vi "USRP-2945-2955 AoA Detection RX Localization using MUSIC.vi"() -> ()   [LabVIEW 2015] (continued)
  out "USRP error out":errorcluster
  out "Queue error out":errorcluster={"status"=TRUE, "code"=1, "source"="Dequeue Element in USRP-2945-2955 AoA Detection RX Localization using MUSIC (manual phase input).vi"}
  out "# elements in queue (it should keep 0)":i32
  out "coerced IQ rate":dbl=1000000.0 format="%#_6p"
  out "coerced carrier frequency":dbl=462651999.98859316 format="%#_6p"
  out "Eigenvalues":cdb[][](array[numeric])=[[1.4802185041005208e-08+5.36819667616762e-26i], [1.1697264580906096e-08+6.7532415852242355e-25i], [1.006365203344385e-08+3.1450001473342563e-25i], [9.127178536995344e-09+1.972647788120172e-25i]]
  out "The number of sources":i32
  out "Ch 1":cdb[](array[numeric])
  out "Ch 2":cdb[](array[numeric])
  out "Ch 3":cdb[](array[numeric])
  out "Ch 4":cdb[](array[numeric])
  in  "Threshold":dbl=0.001
  in  "Filter":string(combo)="IIR"
  in  "Device Name":refnum<k15>="RIO0"
  in  "Gain":dbl=50.0
  in  "Carrier Frequency":dbl=462652000.0 format="%#_6p"
  in  "IQ Rate":dbl=1000000.0 format="%#_6p"
  in  "Samples per Frame":i32=100000
  in  "Samples used":i32=1000
  in  "Stop":bool
  out "Direction":dbl(knob)=54.0 scale=0.0..180.0
  out "MuSIC spectrum":cluster{"Y":dbl[], "Y":dbl[]}[](graph)=[{"Y"=[0.0, 0.5, 1.0, 1.5, 2.0, 2.5, 3.0, 3.5, 4.0, 4.5, 5.0, 5.5, 6.0, 6.5, 7.0, 7.5, 8.0, 8.5, 9.0, 9.5, 10.0, 10.5, 11.0, 11.5, 12.0, 12.5, 13.0, 13.5, 14.0, 14.5, 15.0, 15.5, 16.0, 16.5, 17.0, 17.5, 18.0, 18.5, 19.0, 19.5, 20.0, 20.5, 21.0, 21.5, 22.0, 22.5, 23.0, 23.5, 24.0, 24.5, 25.0, 25.5, 26.0, 26.5, 27.0, 27.5, 28.0, 28.5, 29.0, 29.5, 30.0, 30.5, 31.0, 31.5, 32.0, 32.5, 33.0, 33.5, 34.0, 34.5, 35.0, 35.5, 36.0, 36.5, 37.0, 37.5, 38.0, 38.5, 39.0, 39.5, 40.0, 40.5, 41.0, 41.5, 42.0, 42.5, 43.0, 43.5, 44.0, 44.5, 45.0, 45.5, 46.0, 46.5, 47.0, 47.5, 48.0, 48.5, 49.0, 49.5, 50.0, 50.5, 51.0, 51.5, 52.0, 52.5, 53.0, 53.5, 54.0, 54.5, 55.0, 55.5, 56.0, 56.5, 57.0, 57.5, 58.0, 58.5, 59.0, 59.5, 60.0, 60.5, 61.0, 61.5, 62.0, 62.5, 63.0, 63.5, 64.0, 64.5, 65.0, 65.5, 66.0, 66.5, 67.0, 67.5, 68.0, 68.5, 69.0, 69.5, 70.0, 70.5, 71.0, 71.5, 72.0, 72.5, 73.0, 73.5, 74.0, 74.5, 75.0, 75.5, 76.0, 76.5, 77.0, 77.5, 78.0, 78.5, 79.0, 79.5, 80.0, 80.5, 81.0, 81.5, 82.0, 82.5, 83.0, 83.5, 84.0, 84.5, 85.0, 85.5, 86.0, 86.5, 87.0, 87.5, 88.0, 88.5, 89.0, 89.5, 90.0, 90.5, 91.0, 91.5, 92.0, 92.5, 93.0, 93.5, 94.0, 94.5, 95.0, 95.5, 96.0, 96.5, 97.0, 97.5, 98.0, 98.5, 99.0, 99.5, 100.0, 100.5, 101.0, 101.5, 102.0, 102.5, 103.0, 103.5, 104.0, 104.5, 105.0, 105.5, 106.0, 106.5, 107.0, 107.5, 108.0, 108.5, 109.0, 109.5, 110.0, 110.5, 111.0, 111.5, 112.0, 112.5, 113.0, 113.5, 114.0, 114.5, 115.0, 115.5, 116.0, 116.5, 117.0, 117.5, 118.0, 118.5, 119.0, 119.5, 120.0, 120.5, 121.0, 121.5, 122.0, 122.5, 123.0, 123.5, 124.0, 124.5, 125.0, 125.5, 126.0, 126.5, 127.0, 127.5, 128.0, 128.5, 129.0, 129.5, 130.0, 130.5, 131.0, 131.5, 132.0, 132.5, 133.0, 133.5, 134.0, 134.5, 135.0, 135.5, 136.0, 136.5, 137.0, 137.5, 138.0, 138.5, 139.0, 139.5, 140.0, 140.5, 141.0, 141.5, 142.0, 142.5, 143.0, 143.5, 144.0, 144.5, 145.0, 145.5, 146.0, 146.5, 147.0, 147.5, 148.0, 148.5, 149.0, 149.5, 150.0, 150.5, 151.0, 151.5, 152.0, 152.5, 153.0, 153.5, 154.0, 154.5, 155.0, 155.5, 156.0, 156.5, 157.0, 157.5, 158.0, 158.5, 159.0, 159.5, 160.0, 160.5, 161.0, 161.5, 162.0, 162.5, 163.0, 163.5, 164.0, 164.5, 165.0, 165.5, 166.0, 166.5, 167.0, 167.5, 168.0, 168.5, 169.0, 169.5, 170.0, 170.5, 171.0, 171.5, 172.0, 172.5, 173.0, 173.5, 174.0, 174.5, 175.0, 175.5, 176.0, 176.5, 177.0, 177.5, 178.0, 178.5, 179.0, 179.5, 180.0], "Y"=[-5.811899729347248, -5.811788945154609, -5.811456219896956, -5.810900435008302, -5.810119724458764, -5.809111472133811, -5.807872308183429, -5.806398104359451, -5.80468396836458, -5.802724237241933, -5.8005124698392105, -5.798041438387114, -5.795303119236943, -5.792288682807936, -5.788988482800422, -5.785392044736582, -5.781488053896346, -5.7772643427217965, -5.772707877769499, -5.7678047462961315, -5.762540142569174, -5.756898354000679, -5.750862747208751, -5.744415754118118, -5.737538858218155, -5.730212581103917, -5.722416469433388, -5.7141290824418665, -5.705327980162915, -5.695989712513856, -5.686089809413273, -5.675602772107794, -5.664502065896235, -5.652760114450603, -5.640348295946101, -5.627236941225856, -5.613395334241189, -5.598791715024638, -5.583393285471299, -5.5671662182241946, -5.550075668981941, -5.532085792571921, -5.513159763160277, -5.49325979900109, -5.472347192162216, -5.450382343704117, -5.427324804831905, -5.403133324589545, -5.377765904719838, -5.351179862374778, -5.3233319014288725, -5.294178193223795, -5.26367446765696, -5.231776115620056, -5.198438303897161, -5.163616103746279, -5.127264634514167, -5.08933922377249, -5.049795585614528, -5.008590018916383, -4.965679627544969, -4.921022564687425, -4.874578303682263, -4.826307937950839, -4.776174512857293, -4.72414339256298, -4.6701826651846865, -4.614263589809054, -4.556361089152074, -4.496454291873028, -4.4345271287447865, -4.37056898703177, -4.304575427512951, -4.23654896858595, -4.166499941768175, -4.0944474226349, -4.020420240755714, -3.9444580714556206, -3.866612611169608, -3.7869488367045285, -3.705546346783275, -3.6225007817265817, -3.5379253139230746, -3.451952197738547, -3.36473436261213, -3.2764470271813484, -3.1872893052931306, -3.097485766655833, -3.00728790569245, -2.9169754619790655, -2.826857524730253, -2.7372733425149836, -2.648592748340308, -2.561216100239148, -2.475573629608313, -2.3921240850785184, -2.311352560195529, -2.233767400327271, -2.159896099670763, -2.090280124505112, -2.0254686349572353, -1.9660111247823941, -1.9124490561893586, -1.8653066323675918, -1.825080920372846, -1.792231606160308, -1.7671707253603595, -1.750252760767722, -1.7417655235638205, -1.741922234351378, -1.7508551887582215, -1.7686113303885005, -1.7951499645450042, -1.8303427361424143, -1.8739758740436685, -1.9257545826738764, -1.985309351218376, -2.05220386053326, -2.1259441049219396, -2.2059883135634344, -2.291757254457577, -2.3826445289815563, -2.478026511928559, -2.577271653350932, -2.6797489275454356, -2.7848352846037354, -2.891922025821727, -3.0004200821355216, -3.1097642223873203, -3.2194162547561316, -3.328867310351866, -3.4376393137804877, -3.545285752922436, -3.6513918609080736, -3.7555743190023465, -3.857480581368265, -3.9567879127884336, -4.053202219459528, -4.146456741757979, -4.236310667000184, -4.3225477100838186, -4.404974700736478, -4.48342020802843, -4.5577332258530125, -4.627781937202678, -4.693452570193196, -4.754648354811389, -4.811288586170755, -4.8633077975403225, -4.910655044454052, -4.95329329970793, -4.991198957914255, -5.024361447422167, -5.052782946753302, -5.0764782021732655, -5.095474442561807, -5.109811387302013, -5.119541342430837, -5.124729379733678, -5.125453592781184, -5.121805423057074, -5.113890048274064, -5.101826823687523, -5.085749765663886, -5.065808064920171, -5.042166614708034, -5.015006536768248, -4.984525685143211, -4.950939104940929, -4.914479419955531, -4.875397119761225, -4.833960713642475, -4.790456715681386, -4.745189422721198, -4.698480445040139, -4.6506679487278575, -4.602105569322068, -4.553160958623393, -4.504213931148403, -4.455654183754765, -4.4078785718490305, -4.361287938405952, -4.316283507740531, -4.273262874291828, -4.232615637028488, -4.194718751590697, -4.159931693761562, -4.128591547877956, -4.101008150745145, -4.077459433874929, -4.058187112917876, -4.043392871812516, -4.033235179721314, -4.027826861184281, -4.027233514721177, -4.0314728436793965, -4.040514927394377, -4.054283423074759, -4.0726576518165, -4.095475488291697, -4.122536945130033, -4.153608321461466, -4.188426771499259, -4.2267051436784095, -4.268136943317092, -4.312401281066421, -4.359167684183067, -4.408100666306568, -4.458863972310561, -4.511124436392653, -4.564555412555108, -4.6188397559752, -4.673672350745549, -4.728762193654577, -4.783834054913912, -4.838629745075156, -4.89290902302471, -4.946450183218464, -4.999050361591324, -5.050525599240142, -5.1007107014113, -5.149458926872193, -5.196641539711301, -5.242147252247214, -5.285881584235859, -5.327766160103122, -5.367737962611885, -5.405748558276585, -5.441763307014727, -5.475760565999545, -5.507730895460249, -5.537676272261766, -5.56560931547194, -5.591552526771642, -5.615537547460536, -5.63760443293441, -5.65780094483541, -5.676181860580992, -5.6928082996389175, -5.707747065713711, -5.721070003925492, -5.732853372077691, -5.743177225209535, -5.752124812797417, -5.759781988192395, -5.766236630145941, -5.771578076570148, -5.775896570990074, -5.779282722463007, -5.781826980051599, -5.783619123234026, -5.784747769904936, -5.78529990385665, -5.785360423822333, -5.7850117163045125, -5.784333254497234, -5.7834012256336855, -5.782288189050472, -5.781062767153562, -5.779789371300228, -5.7785279643785605, -5.777333861576134, -5.77625757048852, -5.775344671334597, -5.774635737628531, -5.774166297218368, -5.773966833149636, -5.774062823360696, -5.774474817776394, -5.775218550948578, -5.776305088006599, -5.777741001336681, -5.779528575113503, -5.781666034566305, -5.784147796678896, -5.786964738900682, -5.7901044823838745, -5.793551686259407, -5.797288349517473, -5.801294117163604, -5.805546587472561, -5.810021617353502, -5.814693623064182, -5.819535873762199, -5.8245207756504165, -5.829620144754603, -5.834805466657652, -5.840048141800304, -5.84531971523791, -5.85059209001164, -5.855837723547081, -5.861029806730082, -5.8661424255269115, -5.871150705211694, -5.8760309374378075, -5.880760690541092, -5.8853189035918945, -5.889685964820282, -5.89384377512594, -5.897775797451819, -5.9014670928508375, -5.904904344108733, -5.908075867805808, -5.910971615707127, -5.9135831663665614, -5.91590370781663, -5.917928012194671, -5.919652403128245, -5.921074716669795, -5.922194256534079, -5.923011744352328, -5.9235292656159135, -5.923750211939946, -5.9236792202346, -5.923322109329555, -5.922685814555297, -5.921778320744496, -5.920608594077588, -5.9191865131592145, -5.917522799676668, -5.915628948957734, -5.913517160713805, -5.911200270224418, -5.908691680191939, -5.90600529346939, -5.9031554468409215, -5.900156846012573, -5.897024501951024, -5.89377366868974, -5.890419782705245, -5.886978403951058, -5.883465158623078, -5.879895683717699, -5.876285573432744, -5.872650327451132, -5.869005301138152, -5.865365657675127, -5.861746322144982, -5.85816193757889, -5.8546268229675515, -5.851154933235666, -5.847759821174009, -5.8444546013197485, -5.841251915772633, -5.838163901932055, -5.835202162137941, -5.832377735196798, -5.829701069773007, -5.82718199962475, -5.8248297206633906, -5.822652769815212, -5.820659005664513, -5.818855590857728, -5.817248976248974, -5.815844886768576, -5.814648308997356, -5.813663480431092, -5.812893880421159, -5.812342222779274, -5.812010450036322, -5.811899729347248]}]
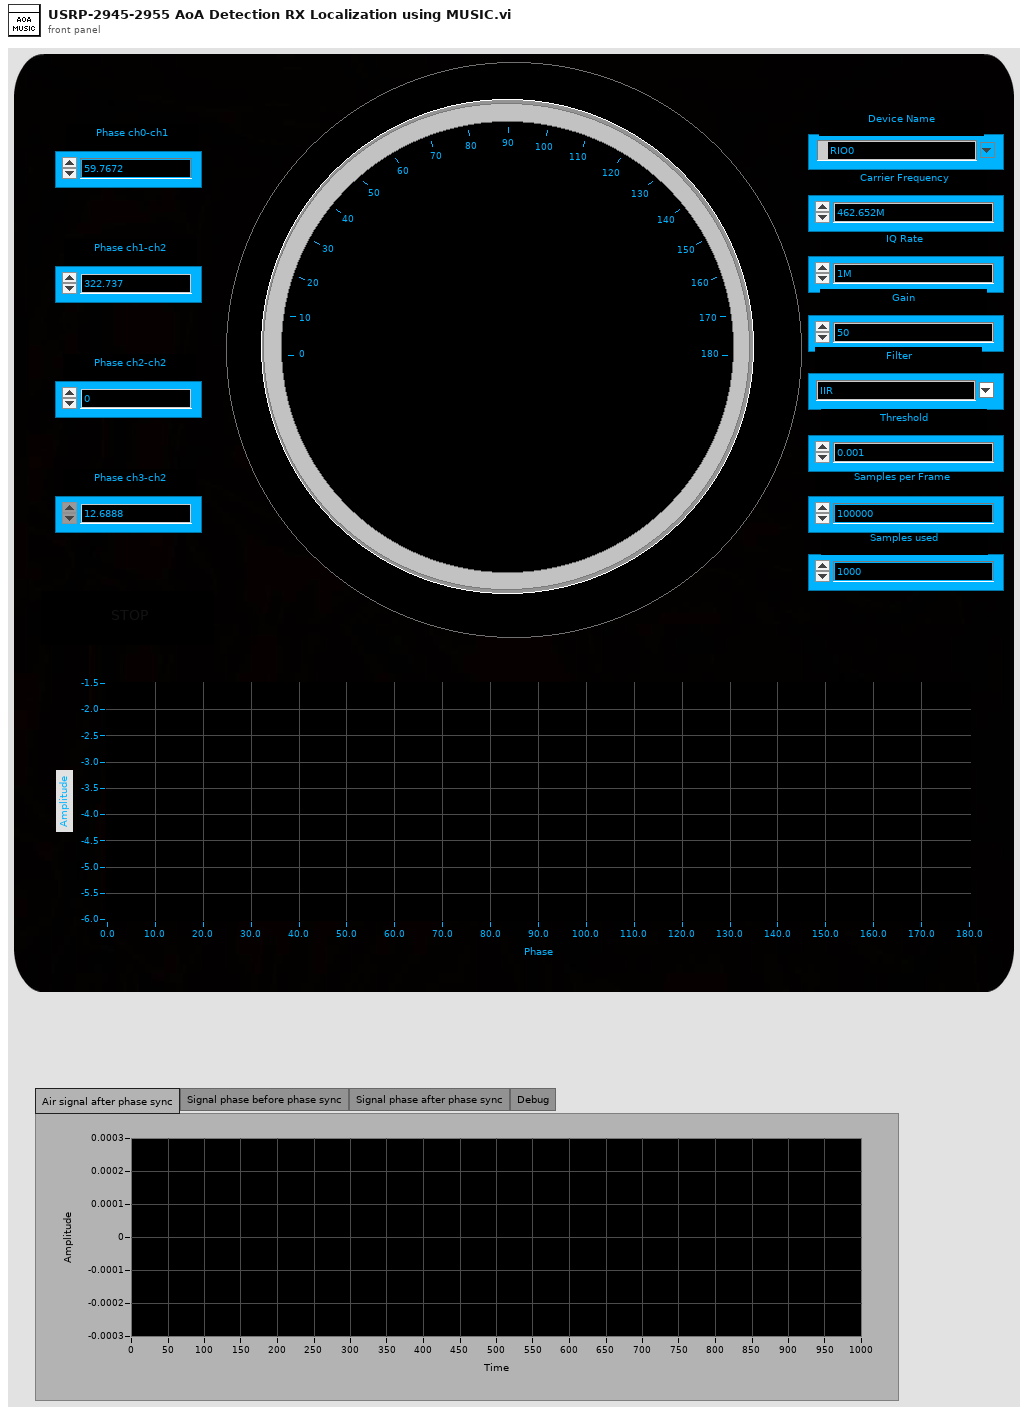
[diagram p1: front panel]
types:
  T1 = enum32{"Air signal after phase sync", "Signal phase before phase sync", "Signal phase after phase sync", "Debug"}
  T2 = typedef "niUSRP Timestamp.ctl" = cluster{"whole seconds":u64, "fractional seconds":dbl}
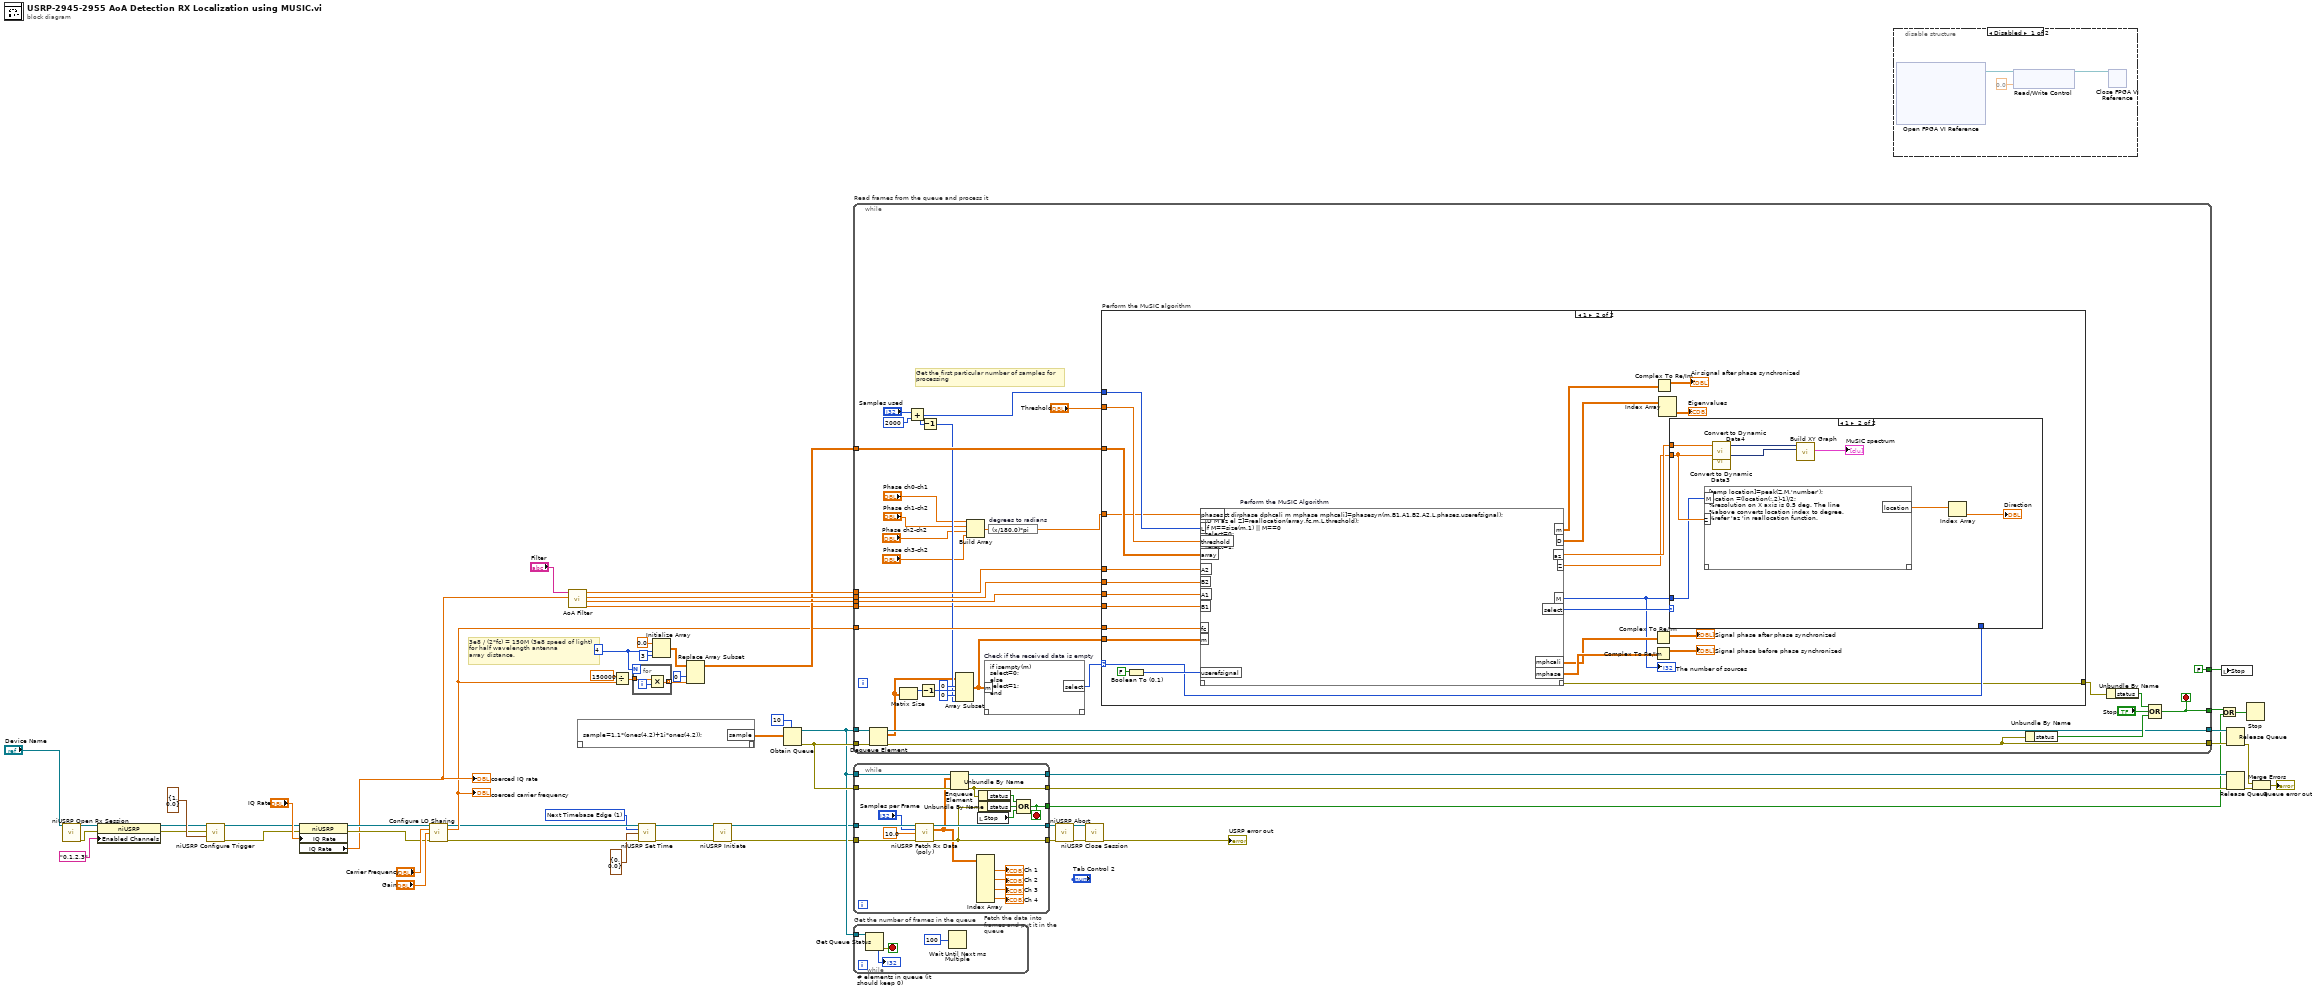
[diagram p0: block diagram]
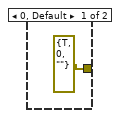
[diagram p3: hidden frame]
diagram:
  w8 = 1 items=["Now", "Next Timebase Edge"] ("apply timestamp")
  w27 = 4
  # "3e8 / (2*fc) = 150M (3e8 speed of light)\nfor half wavelength antenna\narray distance."
  n1 = call <instrlib>:"niUSRP Open Rx Session.vi"("device names"="Device Name") -> ("session handle out"=w26:refnum<k15>, "error out"=w25:errorcluster)  [unwired: 13 in]
  n2 = property class="niUSRP"(reference=w26, error in=w25, "Enabled Channels"="0,1,2,3") -> (reference out=w23:refnum<k15>, error out=w22:errorcluster)
  n3 = call-poly <instrlib>:"niUSRP Configure Trigger.vi"("session handle"=w23, "start trigger time"=T2 {"whole seconds"=1, "fractional seconds"=0.0}, "error in (no error)"=w22) -> ("session handle out"=w6:refnum<k15>, "error out"=w3:errorcluster)  [unwired: 11 in]
  n4 = property class="niUSRP"(reference=w6, error in=w3, "IQ Rate"="IQ Rate") -> (reference out=w16:refnum<k15>, error out=w15:errorcluster, "IQ Rate"=w14:dbl)
  "coerced IQ rate" <- w14
  n5 = call "Configure LO Sharing.vi"("reference"=w16, "Carrier Frequency [Hz]"="Carrier Frequency", "Gain"="Gain", "error in"=w15) -> ("reference out"=w10:refnum<k15>, "Coerced Carrier Frequency"=w13:dbl, "error out"=w12:errorcluster)  [unwired: 9 in]
  "coerced carrier frequency" <- w13
  n6 = call "AoA Filter.vi"("IQ Rate"=w14, "Filter"="Filter") -> ("B1"=w1:dbl[], "A1"=w55:dbl[], "B2"=w54:dbl[], "A2"=w53:dbl[])  [unwired: 6 in]
  n7 = mathscript code="sample=1.1*(ones(4,2)+1i*ones(4,2));"() -> ("sample"=w52:cdb[][])  [unwired: 1 in, 1 out]
  n8 = Divide(x=150000000.0, y=w13) -> (x/y=w35:dbl)
  n9 = for {
    N: w27 -> [_]
    tunnel: w35 -> [w61]
    tunnel: [w60] -> w31 mode=indexing
    i -> [w59]
    n10 = Multiply(x=w61, y=w59) -> (x*y=w60:dbl)
  }
  n11 = call <instrlib>:"niUSRP Set Time.vi"("session handle"=w10, "apply timestamp"=w8, "timestamp"=T2 {"whole seconds"=0, "fractional seconds"=0.0}, "error in (no error)"=w12) -> ("session handle out"=w9:refnum<k15>, "error out"=w11:errorcluster)  [unwired: 10 in]
  n12 = Initialize Array(0.0 ("element"), w27, 3 ("dimension size")) -> (w32:dbl[][])
  n13 = Replace Array Subset(array=w32, new element=w31, index (col)=0 ("disabled index (col)")) -> (w29:dbl[][])  [unwired: 1 in]
  n14 = call <instrlib>:"niUSRP Initiate.vi"("session handle"=w9, "error in (no error)"=w11) -> ("session handle out"=w21:refnum<k15>, "error out"=w20:errorcluster)  [unwired: 12 in]
  n15 = Obtain Queue(max queue size (-1, unlimited)=10, element data type=w52) -> (queue out=w41:refnum<queue>, error out=w42:errorcluster)  [unwired: 3 in, 1 out]
  n16 = while "Read frames from the queue and process it" {
    tunnel: w13 -> [w95]
    tunnel: w29 -> [w94]
    tunnel: [w78] -> w45
    tunnel: [w77] -> w44
    tunnel: w55 -> [w93]
    tunnel: w54 -> [w92]
    tunnel: w53 -> [w91]
    tunnel: w41 -> [w85]
    tunnel: w42 -> [w84]
    tunnel: [w80] -> w38
    tunnel: [FALSE ("Stop")] -> w28
    tunnel: w1 -> [w64]
    stop <- w80 stop-if-true
    # "Get the first particular number of samples for \nprocessing"
    n17 = Dequeue Element(queue=w85, error in (no error)=w84) -> (queue out=w78:refnum<queue>, element=w72:cdb[][], error out=w77:errorcluster)  [unwired: 1 in, 1 out]
    n18 = Matrix Size(0:w72) -> (1:w83:i32)  [unwired: 1 out]
    n19 = Add(x="Samples used", y=2000) -> (x+y=w75:i32)
    n20 = Decrement(x=w83) -> (x-1=w82:i32)
    n21 = Decrement(x=w75) -> (x-1=w74:i32)
    n22 = Array Subset(array=w72, index (row)=0, length (row)=w82, index (col)=0, length (col)=w74) -> (w88:cdb[][])
    n23 = Build Array("Phase ch0-ch1", "Phase ch1-ch2", "Phase ch2-ch2", "Phase ch3-ch2") -> (w66:dbl[])
    n24 = mathscript code="if isempty(m)\nselect=0;\nelse\nselect=1;\nend" "Check if the received data is empty"("m"=w88) -> ("select"=w79:i32)  [unwired: 1 in, 1 out]
    n25 = expression code="(x/180.0)*pi" "degrees to radians"(w66) -> (w71:dbl[])
    n26 = case "Perform the MuSIC algorithm" shown="1" w79 {
      selector: w79 -> [_ w99]
      tunnel: w95 -> [_ w122]
      tunnel: "Threshold" -> [_ w120]
      tunnel: w94 -> [_ w119]
      tunnel: w93 -> [_ w118]
      tunnel: w92 -> [_ w117]
      tunnel: w91 -> [_ w116]
      tunnel: w75 -> [_ w109]
      tunnel: w88 -> [_ w108]
      tunnel: w71 -> [_ w103]
      tunnel: w64 -> [_ w98]
      tunnel: [errorcluster {"status"=TRUE, "code"=0, "source"=""} ("error IO") w97] -> w63
      frame 0, Default {
      }
      frame 1 {
        n27 = Boolean To (0,1)(Boolean=FALSE ("Userefsignal for phase \nsync")) -> (0, 1=w102:i16)
        n28 = mathscript code="[L direct dirphase dphcali m mphase mphcali]=phasesyn(m,B1,A1,B2,A2,L,phases,userefsignal);\n[D M az el Z]=reallocation(array,fc,m,L,threshold);\nif M==size(m,1) || M==0 \nselect=0;\nelse\nselect=1;\nend" "Perform the MuSIC Algorithm"("m"=w108, "fc"=w122, "L"=w109, "array"=w119, "threshold"=w120, "B1"=w98, "A1"=w118, "B2"=w117, "A2"=w116, "phases"=w103, "userefsignal"=w102) -> ("??"=w97:errorcluster, "D"=w121:cdb[][], "az"=w107:dbl[], "Z"=w106:cdb[], "M"=w104:i32, "m"=w115:cdb[][], "mphase"=w111:dbl[][], "mphcali"=w110:dbl[][], "select"=w105:i32)  [unwired: 1 in]
        "The number of sources" <- w104
        n29 = Complex To Re/Im(x + iy=w110) -> (x=→"Signal phase after phase synchronized":dbl[][])  [unwired: 1 out]
        n30 = Complex To Re/Im(x + iy=w111) -> (x=→"Signal phase before phase synchronized":dbl[][])  [unwired: 1 out]
        n31 = Complex To Re/Im(x + iy=w115) -> (x=→"Air signal after phase synchronized":dbl[][])  [unwired: 1 out]
        n32 = Index Array(array=w121) -> (element=→"Eigenvalues":cdb[][])  [unwired: 2 in]
        n33 = case shown="1" w105 {
          tunnel: w107 -> [_ w127]
          tunnel: w106 -> [_ w126]
          tunnel: w104 -> [_ w125]
          tunnel: w99 -> [_ _]
          frame 0, Default {
          }
          frame 1 {
            n34 = mathscript code="[temp location]=peak(Z,M,'number');\nlocation =(location(:,2)-1)/2;\n%resolution on X axis is 0.5 deg. The line\n%above converts location index to degree.\n%refer 'az 'in reallocation function."("M"=w125, "Z"=w126) -> ("location"=w124:dbl[])  [unwired: 1 in, 1 out]
            n35 = call "Convert to Dynamic Data4"("Array"=w127) -> ("Dynamic Data Type"=w129:dynamicdata)  [unwired: 3 in]
            n36 = call "Convert to Dynamic Data3"("Array"=w126) -> ("Dynamic Data Type"=w128:dynamicdata)  [unwired: 3 in]
            n37 = call "Build XY Graph"("Y Input"=w128, "X Input"=w129) -> ("XY Graph"=→"MuSIC spectrum":cluster{"Y":dbl[], "Y":dbl[]}[])  [unwired: 3 in, 6 out]
            n38 = Index Array(array=w124) -> (element=→"Direction":dbl)  [unwired: 1 in]
          }
        }
      }
    }
    n39 = Unbundle By Name(w77) -> ("status"=w81:bool)
    n40 = Unbundle By Name(w63) -> ("status"=w62:bool)
    n41 = Compound Arithmetic op=OR(w62, "Stop", w81) -> (w80:bool)
  }
  n42 = while "Fetch the data into frames and put it in the queue" {
    tunnel: w21 -> [w148]
    tunnel: w20 -> [w147]
    tunnel: w41 -> [w146]
    tunnel: w42 -> [w145]
    tunnel: [w144] -> w47
    tunnel: [w141] -> w46
    tunnel: [w143] -> w50
    tunnel: [w142] -> w49
    tunnel: [w136] -> w37
    stop <- w136 stop-if-true
    n43 = call-poly <instrlib>:"niUSRP Fetch Rx Data (poly).vi"("session handle"=w148, "number of samples"="Samples per Frame", "timeout"=10.0, "error in (no error)"=w147) -> ("session handle out"=w143:refnum<k15>, "data"=w135:cdb[][], "error out"=w142:errorcluster)  [unwired: 8 in, 1 out]
    n44 = Enqueue Element(queue=w146, element=w135, error in (no error)=w145) -> (queue out=w144:refnum<queue>, error out=w141:errorcluster)  [unwired: 1 in, 1 out]
    n45 = Index Array(array=w135) -> (element #1=→"Ch 1":cdb[], element #2=→"Ch 2":cdb[], element #3=→"Ch 3":cdb[], element #4=→"Ch 4":cdb[])  [unwired: 8 in]
    n46 = local read "Stop"() -> (w137:bool)
    n47 = Unbundle By Name(w141) -> ("status"=w139:bool)
    n48 = Unbundle By Name(w142) -> ("status"=w138:bool)
    n49 = Compound Arithmetic op=OR(w139, w138, w137) -> (w136:bool)
  }
  n50 = while "Get the number of frames in the queue" {
    tunnel: w41 -> [w153]
    stop <- w151 stop-if-true
    n51 = Get Queue Status(queue=w153) -> (error out=w151:errorcluster, # elements in queue=→"# elements in queue (it should keep 0)":i32)  [unwired: 2 in, 6 out]
    n52 = Wait Until Next ms Multiple(millisecond multiple=100) -> ()  [unwired: 1 out]
  }
  n53 = call <instrlib>:"niUSRP Abort.vi"("session handle"=w50, "error in (no error)"=w49) -> ("session handle out"=w58:refnum<k15>, "error out"=w57:errorcluster)  [unwired: 12 in]
  n54 = call <instrlib>:"niUSRP Close Session.vi"("session handle"=w58, "error in (no error)"=w57) -> ("error out"=→"USRP error out":errorcluster)  [unwired: 13 in]
  n55 = disable-structure shown="Disabled" {
    frame Disabled {
      n56 = xnode "Open FPGA VI Reference"() -> ("FPGA VI Reference Out"=w155:refnum<k20>)  [unwired: 2 in, 1 out]
      n57 = xnode "Read/Write Control"("FPGA VI Reference In"=w155, "Direction Value"=sgl 0.0) -> ("FPGA VI Reference Out"=w156:refnum<k20>)  [unwired: 1 in, 1 out]
      n58 = xnode "Close FPGA VI Reference"("FPGA VI Reference In"=w156) -> ()  [unwired: 1 in, 1 out]
    }
    frame Enabled {
    }
  }
  n59 = Or(x=w38, y=w37) -> (x .or. y?=w43:bool)
  n60 = local write "Stop"(w28) -> ()
  n61 = Release Queue(queue=w45, error in (no error)=w44) -> (error out=w39:errorcluster)  [unwired: 1 in, 2 out]
  n62 = Release Queue(queue=w47, error in (no error)=w46) -> (error out=w40:errorcluster)  [unwired: 1 in, 2 out]
  n63 = Stop(stop? (T)=w43) -> ()
  n64 = Merge Errors(w39, w40) -> (→"Queue error out":errorcluster)
